vi "FlexMag - 24-03-2023.vi"() -> ()   [LabVIEW 2018] (continued)
            n18652 = local write "CH2_Motor DO"(w23090) -> ()
            n18653 = local write "CH3_Motor DO"(w23090) -> ()
            n18654 = local write "CH4_Motor DO"(w23090) -> ()
            n18655 = local write "step count"(0.0 ("step count")) -> ()
            n18656 = local write "forward roll"(FALSE ("forward roll")) -> ()
            n18657 = Wait (ms)(milliseconds to wait=u32 300) -> ()  [unwired: 1 out]
          }
        }
      }
      frame 2 {
        # "backward roll"
        n18658 = stacked-sequence {
          tunnel: w23093 -> [w23094 _ _ _ _ _ w23153 w23163 _]
          frame #0 {
            n18659 = Wait (ms)(milliseconds to wait=u32 100) -> ()  [unwired: 1 out]
            n18660 = case shown="0, Default" w23094 {
              frame 0, Default {
                n18661 = local write "roll error"(TRUE ("roll error")) -> ()
                n18662 = local write "Warning Message"("Choose Cassette Position !" ("Warning Message")) -> ()
                n18663 = Wait (ms)(milliseconds to wait=u32 100) -> ()  [unwired: 1 out]
              }
              frame 1 {
                n18664 = local read "CH1_SRV1_Piston_For_DI"() -> (w23099:bool)
                n18665 = case shown="False" w23099 {
                  frame False {
                    n18666 = local write "roll error"(TRUE ("roll error")) -> ()
                    n18667 = Wait (ms)(milliseconds to wait=u32 100) -> ()  [unwired: 1 out]
                  }
                  frame True {
                  }
                }
              }
              frame 2 {
                n18668 = local read "CH2_SRV1_Piston_For_DI"() -> (w23102:bool)
                n18669 = case shown="False" w23102 {
                  frame False {
                    n18670 = local write "roll error"(TRUE ("roll error")) -> ()
                    n18671 = Wait (ms)(milliseconds to wait=u32 100) -> ()  [unwired: 1 out]
                  }
                  frame True {
                  }
                }
              }
              frame 3 {
                n18672 = local read "CH3_SRV1_Piston_For_DI"() -> (w23105:bool)
                n18673 = case shown="False" w23105 {
                  frame False {
                    n18674 = local write "roll error"(TRUE ("roll error")) -> ()
                    n18675 = Wait (ms)(milliseconds to wait=u32 100) -> ()  [unwired: 1 out]
                  }
                  frame True {
                  }
                }
              }
              frame 4 {
                n18676 = local read "CH4_SRV1_Piston_For_DI"() -> (w23108:bool)
                n18677 = case shown="False" w23108 {
                  frame False {
                    n18678 = local write "roll error"(TRUE ("roll error")) -> ()
                    n18679 = Wait (ms)(milliseconds to wait=u32 100) -> ()  [unwired: 1 out]
                  }
                  frame True {
                  }
                }
              }
            }
          }
          frame #1 {
            n18680 = flat-sequence {
              frame #0 {
                n18681 = local write "Roll Forw"(FALSE ("Roll Forw")) -> ()
              }
              frame #1 {
                n18682 = Wait (ms)(milliseconds to wait=u32 300) -> ()  [unwired: 1 out]
              }
              frame #2 {
                n18683 = local write "TC parameter set"(TRUE ("TC parameter set")) -> ()
              }
              frame #3 {
                n18684 = Wait (ms)(milliseconds to wait=u32 300) -> ()  [unwired: 1 out]
              }
            }
            n18685 = disable-structure shown="Disabled" {
              frame Disabled {
                n18686 = local read "lap number right actual"() -> (w23114:dbl)
                n18687 = local write "lap number left target"(w23114) -> ()
              }
              frame Enabled {
              }
            }
            n18688 = local write "lap number left actual"(0.0 ("lap number left actual")) -> ()
            n18689 = local write "lap number right actual"(0.0 ("lap number left actual")) -> ()
            n18690 = local read "step count"() -> (w23112:dbl)
            n18691 = local write "step count 2"(w23112) -> ()
          }
          frame #2 {
            n18692 = local read "back roll"() -> (w23119:bool)
            n18693 = case shown="True" w23119 {
              frame False {
              }
              frame True {
                n18694 = while {
                  i -> [w23125]
                  stop <- w23123 stop-if-true
                  n18695 = Wait Until Next ms Multiple(millisecond multiple=u32 300) -> ()  [unwired: 1 out]
                  n18696 = local read "TC parameter set"() -> (w23129:bool)
                  n18697 = local read "back roll"() -> (w23121:bool)
                  n18698 = local read "ABORT"() -> (w23127:bool)
                  n18699 = Not(x=w23129) -> (.not. x?=w23126:bool)
                  n18700 = Not(x=w23121) -> (.not. x?=w23120:bool)
                  n18701 = Greater Or Equal?(x=w23125, y=u32 400 ("millisecond multiple")) -> (x >= y?=w23122:bool)
                  n18702 = Compound Arithmetic op=OR(w23122, w23126, w23127, w23120) -> (w23123:bool)
                  n18703 = local write "roll error"(w23122) -> ()
                }
              }
            }
          }
          frame #3 {
            n18704 = local read "back roll"() -> (w23130:bool)
            n18705 = case shown="True" w23130 {
              frame False {
              }
              frame True {
                n18706 = flat-sequence {
                  frame #0 {
                    n18707 = disable-structure shown="Enabled" {
                      disable-tunnel: [w23134 sgl 0.1 ("TC1_overspeed_value")] -> w23131
                      frame Disabled {
                        n18708 = local read "output_pid"() -> (w23134:dbl)
                      }
                      frame Enabled {
                      }
                    }
                    n18709 = local read "tension value"() -> (w23133:dbl)
                    n18710 = local write "TC2_set_value"(w23133) -> ()
                    n18711 = local write "TC1_overspeed_value"(w23131) -> ()
                    n18712 = local write "current voltage"(w23131) -> ()
                    n18713 = Wait (ms)(milliseconds to wait=u32 1000) -> ()  [unwired: 1 out]
                  }
                  frame #1 {
                    n18714 = local write "TC1_overspeed_set"(TRUE ("TC2 Set moxa")) -> ()
                    n18715 = local write "TC2_auto_set"(TRUE ("TC1_set")) -> ()
                  }
                  frame #2 {
                    n18716 = local write "TC2_overspeed_value"(sgl 0.0 ("TC2_set_value")) -> ()
                    n18717 = local write "TC1_set_value"(sgl 0.0 ("TC2_set_value")) -> ()
                    n18718 = Wait (ms)(milliseconds to wait=u32 2000) -> ()  [unwired: 1 out]
                  }
                  frame #3 {
                    n18719 = local write "TC2_overspeed_set"(TRUE ("TC2_auto_set")) -> ()
                    n18720 = local write "TC1_auto_set"(TRUE ("TC2_auto_set")) -> ()
                  }
                }
              }
            }
          }
          frame #4 {
            n18721 = local read "back roll"() -> (w23143:bool)
            n18722 = case shown="True" w23143 {
              frame False {
              }
              frame True {
                n18723 = flat-sequence {
                  frame #0 {
                    w23145 = FALSE ("CH1_SRV_Direction_Clockwise_DO")
                    n18724 = Wait (ms)(milliseconds to wait=u32 100) -> ()  [unwired: 1 out]
                    n18725 = local write "CH1_SRV_Direction_Clockwise_DO"(w23145) -> ()
                    n18726 = local write "CH2_SRV_Direction_Clockwise_DO"(w23145) -> ()
                    n18727 = local write "CH3_SRV_Direction_Clockwise_DO"(w23145) -> ()
                    n18728 = local write "CH4_SRV_Direction_Clockwise_DO"(w23145) -> ()
                    n18729 = disable-structure shown="Disabled" {
                      frame Disabled {
                        n18730 = local write "setpoint"(0.1 ("setpoint")) -> ()
                      }
                      frame Enabled {
                      }
                    }
                  }
                  frame #1 {
                    n18731 = Wait (ms)(milliseconds to wait=u32 3000) -> ()  [unwired: 1 out]
                  }
                }
              }
            }
          }
          frame #5 {
            n18732 = local read "back roll"() -> (w23148:bool)
            n18733 = case shown="True" w23148 {
              frame False {
              }
              frame True {
                n18734 = disable-structure shown="Disabled" {
                  frame Disabled {
                    w23151 = 0.1 ("lower limit")
                    n18735 = Bundle("lower limit"=w23151, "lower limit"=w23151) -> (w23152:cluster{"lower limit":dbl, "lower limit":dbl})  [unwired: 1 in]
                    n18736 = local write "output range"(w23152) -> ()
                  }
                  frame Enabled {
                  }
                }
                n18737 = local write "Tension_Controllers_Start/Stop DO"(TRUE ("CH1_SRV_Direction_Clockwise_DO")) -> ()
                n18738 = Wait (ms)(milliseconds to wait=u32 100) -> ()  [unwired: 1 out]
              }
            }
          }
          frame #6 {
            n18739 = local read "back roll"() -> (w23154:bool)
            n18740 = case shown="True" w23154 {
              tunnel: w23153 -> [_ w23157]
              frame False {
              }
              frame True {
                n18741 = case shown="1" w23157 {
                  frame 0, Default {
                    n18742 = local write "roll error"(TRUE ("roll error")) -> ()
                  }
                  frame 1 {
                    n18743 = local write "CH1_Motor DO"(TRUE ("CH1_Motor DO")) -> ()
                  }
                  frame 2 {
                    n18744 = local write "CH2_Motor DO"(TRUE ("CH1_Motor DO")) -> ()
                  }
                  frame 3 {
                    n18745 = local write "CH3_Motor DO"(TRUE ("CH1_Motor DO")) -> ()
                  }
                  frame 4 {
                    n18746 = local write "CH4_Motor DO"(TRUE ("CH1_Motor DO")) -> ()
                  }
                }
                n18747 = local write "QR continuous mode"(TRUE ("QR continuous mode")) -> ()
                n18748 = local write "pid output"(TRUE ("pid output")) -> ()
              }
            }
          }
          frame #7 {
            n18749 = local read "back roll"() -> (w23164:bool)
            n18750 = case shown="True" w23164 {
              tunnel: w23163 -> [_ w23165]
              frame False {
              }
              frame True {
                n18751 = case shown="4" w23165 {
                  frame 0, Default {
                    n18752 = local write "roll error"(TRUE ("roll error")) -> ()
                  }
                  frame 1 {
                    n18753 = while {
                      i -> [w23187]
                      stop <- w23197 stop-if-true
                      n18754 = local read "CH1_SRV2_COUNTER_DI"() -> (w23193:bool)
                      n18755 = local read "Ch1_srv1_counter DI"() -> (w23185:bool)
                      n18756 = Wait Until Next ms Multiple(millisecond multiple=u32 100) -> ()  [unwired: 1 out]
                      n18757 = Greater Or Equal?(x=w23187, y=200) -> (x >= y?=w23188:bool)
                      n18758 = feedback #330() -> (w23194:bool)  [unwired: 1 in]
                      n18759 = feedback-in #330(w23193) -> ()
                      n18760 = feedback #331() -> (w23184:bool)  [unwired: 1 in]
                      n18761 = feedback-in #331(w23185) -> ()
                      n18762 = case shown="True" w23188 {
                        tunnel: [FALSE ("backroll stop cmd") w23204] -> w23190
                        frame False {
                        }
                        frame True {
                          n18763 = local read "backroll stop cmd"() -> (w23204:bool)
                        }
                      }
                      n18764 = Implies(1:w23193, 2:w23194) -> (0:w23195:bool)
                      n18765 = Implies(1:w23185, 2:w23184) -> (0:w23183:bool)
                      n18766 = Not(x=w23195) -> (.not. x?=w23192:bool)
                      n18767 = Not(x=w23183) -> (.not. x?=w23182:bool)
                      n18768 = local read "max rotation number"() -> (w23177:dbl)
                      n18769 = case shown="True" w23192 {
                        frame False {
                        }
                        frame True {
                          n18770 = local read "output range"() -> (w23205:cluster{"output high":dbl, "output low":dbl})
                          n18771 = local read "lap number right actual"() -> (w23212:dbl)
                          n18772 = Unbundle By Name(w23205) -> ("output high"=w23207:dbl, "output low"=w23210:dbl)
                          n18773 = Increment(x=w23212) -> (x+1=w23211:dbl)
                          n18774 = local read "decreasing voltage"() -> (w23206:dbl)
                          n18775 = local write "lap number right actual"(w23211) -> ()
                          n18776 = Subtract(x=w23207, y=w23206) -> (x-y=w23209:dbl)
                          n18777 = Bundle(w23209, "output low"=w23210) -> (w23208:cluster{dbl, "output low":dbl})  [unwired: 1 in]
                          n18778 = local write "output range"(w23208) -> ()
                        }
                      }
                      n18779 = case shown="True" w23182 {
                        frame False {
                        }
                        frame True {
                          n18780 = local read "lap number left actual"() -> (w23202:dbl)
                          n18781 = Increment(x=w23202) -> (x+1=w23201:dbl)
                          n18782 = local write "lap number left actual"(w23201) -> ()
                        }
                      }
                      n18783 = local read "lap number right actual"() -> (w23186:dbl)
                      n18784 = local read "lap number left actual"() -> (w23181:dbl)
                      n18785 = local read "abort ch1"() -> (w23191:bool)
                      n18786 = local read "back roll"() -> (w23200:bool)
                      n18787 = Greater Or Equal?(x=w23181, y=w23177) -> (x >= y?=w23179:bool)
                      n18788 = Greater Or Equal?(x=w23186, y=w23177) -> (x >= y?=w23180:bool)
                      n18789 = Not(x=w23200) -> (.not. x?=w23199:bool)
                      n18790 = Or(x=w23180, y=w23179) -> (x .or. y?=w23178:bool)
                      n18791 = Compound Arithmetic op=OR(w23191, w23199, w23190, w23178) -> (w23197:bool)
                      n18792 = Not(x=w23197) -> (.not. x?=w23198:bool)
                      n18793 = local write "CH1_Motor DO"(w23198) -> ()
                    }
                    n18794 = while {
                      stop <- w23173 stop-if-true
                      n18795 = stacked-sequence {
                        frame #0 {
                          n18796 = local read "output_pid"() -> (w23174:dbl)
                          n18797 = Wait (ms)(milliseconds to wait=u32 25) -> ()  [unwired: 1 out]
                          n18798 = local write "TC1_overspeed_value"(w23174) -> ()
                          n18799 = local write "current voltage"(w23174) -> ()
                        }
                        frame #1 {
                          n18800 = local write "TC1_overspeed_set"(TRUE ("TC2_overspeed_set")) -> ()
                        }
                      }
                      n18801 = local read "CH1_Motor DO"() -> (w23168:bool)
                      n18802 = local read "back roll"() -> (w23171:bool)
                      n18803 = local read "set speed (ms)"() -> (w23169:u32)
                      n18804 = local read "abort ch1"() -> (w23172:bool)
                      n18805 = Not(x=w23171) -> (.not. x?=w23170:bool)
                      n18806 = Not(x=w23168) -> (.not. x?=w23167:bool)
                      n18807 = Compound Arithmetic op=OR(w23167, w23172, w23170) -> (w23173:bool)
                      n18808 = Wait Until Next ms Multiple(millisecond multiple=w23169) -> ()  [unwired: 1 out]
                    }
                  }
                  frame 2 {
                    n18809 = while {
                      i -> [w23234]
                      stop <- w23243 stop-if-true
                      n18810 = local read "CH2_SRV2_COUNTER_DI"() -> (w23239:bool)
                      n18811 = Greater Or Equal?(x=w23234, y=200) -> (x >= y?=w23233:bool)
                      n18812 = case shown="True" w23233 {
                        tunnel: [FALSE ("backroll stop cmd") w23250] -> w23236
                        frame False {
                        }
                        frame True {
                          n18813 = local read "backroll stop cmd"() -> (w23250:bool)
                        }
                      }
                      n18814 = local read "Ch2_srv1_counter DI"() -> (w23228:bool)
                      n18815 = feedback #332() -> (w23240:bool)  [unwired: 1 in]
                      n18816 = feedback-in #332(w23239) -> ()
                      n18817 = Implies(1:w23239, 2:w23240) -> (0:w23241:bool)
                      n18818 = Not(x=w23241) -> (.not. x?=w23238:bool)
                      n18819 = local read "max rotation number"() -> (w23223:dbl)
                      n18820 = case shown="True" w23238 {
                        frame False {
                        }
                        frame True {
                          n18821 = local read "lap number right actual"() -> (w23258:dbl)
                          n18822 = local read "output range"() -> (w23251:cluster{"output high":dbl, "output low":dbl})
                          n18823 = Unbundle By Name(w23251) -> ("output high"=w23253:dbl, "output low"=w23256:dbl)
                          n18824 = Increment(x=w23258) -> (x+1=w23257:dbl)
                          n18825 = local write "lap number right actual"(w23257) -> ()
                          n18826 = local read "decreasing voltage"() -> (w23252:dbl)
                          n18827 = Subtract(x=w23253, y=w23252) -> (x-y=w23255:dbl)
                          n18828 = Bundle(w23255, "output low"=w23256) -> (w23254:cluster{dbl, "output low":dbl})  [unwired: 1 in]
                          n18829 = local write "output range"(w23254) -> ()
                        }
                      }
                      n18830 = feedback #333() -> (w23229:bool)  [unwired: 1 in]
                      n18831 = feedback-in #333(w23228) -> ()
                      n18832 = Implies(1:w23228, 2:w23229) -> (0:w23230:bool)
                      n18833 = Not(x=w23230) -> (.not. x?=w23231:bool)
                      n18834 = local read "lap number right actual"() -> (w23232:dbl)
                      n18835 = case shown="True" w23231 {
                        frame False {
                        }
                        frame True {
                          n18836 = local read "lap number left actual"() -> (w23248:dbl)
                          n18837 = Increment(x=w23248) -> (x+1=w23247:dbl)
                          n18838 = local write "lap number left actual"(w23247) -> ()
                        }
                      }
                      n18839 = local read "lap number left actual"() -> (w23227:dbl)
                      n18840 = Greater Or Equal?(x=w23232, y=w23223) -> (x >= y?=w23226:bool)
                      n18841 = local read "abort ch2"() -> (w23237:bool)
                      n18842 = local read "back roll"() -> (w23246:bool)
                      n18843 = Greater Or Equal?(x=w23227, y=w23223) -> (x >= y?=w23225:bool)
                      n18844 = Or(x=w23226, y=w23225) -> (x .or. y?=w23224:bool)
                      n18845 = Not(x=w23246) -> (.not. x?=w23245:bool)
                      n18846 = Compound Arithmetic op=OR(w23237, w23245, w23236, w23224) -> (w23243:bool)
                      n18847 = Not(x=w23243) -> (.not. x?=w23244:bool)
                      n18848 = local write "CH2_Motor DO"(w23244) -> ()
                      n18849 = Wait Until Next ms Multiple(millisecond multiple=u32 100) -> ()  [unwired: 1 out]
                    }
                    n18850 = while {
                      stop <- w23219 stop-if-true
                      n18851 = stacked-sequence {
                        frame #0 {
                          n18852 = local read "output_pid"() -> (w23220:dbl)
                          n18853 = Wait (ms)(milliseconds to wait=u32 25) -> ()  [unwired: 1 out]
                          n18854 = local write "TC1_overspeed_value"(w23220) -> ()
                          n18855 = local write "current voltage"(w23220) -> ()
                        }
                        frame #1 {
                          n18856 = local write "TC1_overspeed_set"(TRUE ("TC2_overspeed_set")) -> ()
                        }
                      }
                      n18857 = local read "CH2_Motor DO"() -> (w23214:bool)
                      n18858 = local read "back roll"() -> (w23217:bool)
                      n18859 = local read "set speed (ms)"() -> (w23215:u32)
                      n18860 = local read "abort ch2"() -> (w23218:bool)
                      n18861 = Not(x=w23217) -> (.not. x?=w23216:bool)
                      n18862 = Not(x=w23214) -> (.not. x?=w23213:bool)
                      n18863 = Compound Arithmetic op=OR(w23213, w23218, w23216) -> (w23219:bool)
                      n18864 = Wait Until Next ms Multiple(millisecond multiple=w23215) -> ()  [unwired: 1 out]
                    }
                  }
                  frame 3 {
                    n18865 = while {
                      i -> [w23284]
                      stop <- w23279 stop-if-true
                      n18866 = local read "CH3_SRV2_COUNTER_DI"() -> (w23287:bool)
                      n18867 = Greater Or Equal?(x=w23284, y=200) -> (x >= y?=w23283:bool)
                      n18868 = case shown="True" w23283 {
                        tunnel: [FALSE ("backroll stop cmd") w23296] -> w23280
                        frame False {
                        }
                        frame True {
                          n18869 = local read "backroll stop cmd"() -> (w23296:bool)
                        }
                      }
                      n18870 = feedback #334() -> (w23288:bool)  [unwired: 1 in]
                      n18871 = feedback-in #334(w23287) -> ()
                      n18872 = local read "Ch3_srv1_counter DI"() -> (w23277:bool)
                      n18873 = Implies(1:w23287, 2:w23288) -> (0:w23289:bool)
                      n18874 = Not(x=w23289) -> (.not. x?=w23286:bool)
                      n18875 = case shown="True" w23286 {
                        frame False {
                        }
                        frame True {
                          n18876 = local read "output range"() -> (w23302:cluster{"output high":dbl, "output low":dbl})
                          n18877 = local read "lap number right actual"() -> (w23304:dbl)
                          n18878 = Unbundle By Name(w23302) -> ("output high"=w23300:dbl, "output low"=w23297:dbl)
                          n18879 = Increment(x=w23304) -> (x+1=w23303:dbl)
                          n18880 = local read "decreasing voltage"() -> (w23301:dbl)
                          n18881 = local write "lap number right actual"(w23303) -> ()
                          n18882 = Subtract(x=w23300, y=w23301) -> (x-y=w23298:dbl)
                          n18883 = Bundle(w23298, "output low"=w23297) -> (w23299:cluster{dbl, "output low":dbl})  [unwired: 1 in]
                          n18884 = local write "output range"(w23299) -> ()
                        }
                      }
                      n18885 = local read "max rotation number"() -> (w23269:dbl)
                      n18886 = local read "lap number right actual"() -> (w23278:dbl)
                      n18887 = feedback #335() -> (w23276:bool)  [unwired: 1 in]
                      n18888 = feedback-in #335(w23277) -> ()
                      n18889 = Implies(1:w23277, 2:w23276) -> (0:w23275:bool)
                      n18890 = Not(x=w23275) -> (.not. x?=w23274:bool)
                      n18891 = case shown="True" w23274 {
                        frame False {
                        }
                        frame True {
                          n18892 = local read "lap number left actual"() -> (w23294:dbl)
                          n18893 = Increment(x=w23294) -> (x+1=w23293:dbl)
                          n18894 = local write "lap number left actual"(w23293) -> ()
                        }
                      }
                      n18895 = local read "lap number left actual"() -> (w23273:dbl)
                      n18896 = Greater Or Equal?(x=w23278, y=w23269) -> (x >= y?=w23271:bool)
                      n18897 = local read "abort ch3"() -> (w23282:bool)
                      n18898 = local read "back roll"() -> (w23292:bool)
                      n18899 = Greater Or Equal?(x=w23273, y=w23269) -> (x >= y?=w23272:bool)
                      n18900 = Not(x=w23292) -> (.not. x?=w23281:bool)
                      n18901 = Or(x=w23271, y=w23272) -> (x .or. y?=w23270:bool)
                      n18902 = Compound Arithmetic op=OR(w23282, w23281, w23280, w23270) -> (w23279:bool)
                      n18903 = Not(x=w23279) -> (.not. x?=w23291:bool)
                      n18904 = local write "CH3_Motor DO"(w23291) -> ()
                      n18905 = Wait Until Next ms Multiple(millisecond multiple=u32 100) -> ()  [unwired: 1 out]
                    }
                    n18906 = while {
                      stop <- w23265 stop-if-true
                      n18907 = stacked-sequence {
                        frame #0 {
                          n18908 = local read "output_pid"() -> (w23266:dbl)
                          n18909 = Wait (ms)(milliseconds to wait=u32 25) -> ()  [unwired: 1 out]
                          n18910 = local write "TC1_overspeed_value"(w23266) -> ()
                          n18911 = local write "current voltage"(w23266) -> ()
                        }
                        frame #1 {
                          n18912 = local write "TC1_overspeed_set"(TRUE ("TC2_overspeed_set")) -> ()
                        }
                      }
                      n18913 = local read "CH3_Motor DO"() -> (w23260:bool)
                      n18914 = local read "back roll"() -> (w23263:bool)
                      n18915 = local read "set speed (ms)"() -> (w23261:u32)
                      n18916 = local read "abort ch3"() -> (w23264:bool)
                      n18917 = Not(x=w23263) -> (.not. x?=w23262:bool)
                      n18918 = Not(x=w23260) -> (.not. x?=w23259:bool)
                      n18919 = Compound Arithmetic op=OR(w23259, w23264, w23262) -> (w23265:bool)
                      n18920 = Wait Until Next ms Multiple(millisecond multiple=w23261) -> ()  [unwired: 1 out]
                    }
                  }
                  frame 4 {
                    n18921 = while {
                      i -> [w23325]
                      stop <- w23335 stop-if-true
                      n18922 = local read "CH4_SRV2_COUNTER_DI"() -> (w23331:bool)
                      n18923 = feedback #336() -> (w23332:bool)  [unwired: 1 in]
                      n18924 = feedback-in #336(w23331) -> ()
                      n18925 = local read "Ch4_srv1_counter DI"() -> (w23321:bool)
                      n18926 = Implies(1:w23331, 2:w23332) -> (0:w23333:bool)
                      n18927 = Not(x=w23333) -> (.not. x?=w23330:bool)
                      n18928 = Greater Or Equal?(x=w23325, y=200) -> (x >= y?=w23326:bool)
                      n18929 = case shown="True" w23330 {
                        frame False {
                        }
                        frame True {
                          n18930 = local read "output range"() -> (w23348:cluster{"output high":dbl, "output low":dbl})
                          n18931 = local read "lap number right actual"() -> (w23350:dbl)
                          n18932 = Unbundle By Name(w23348) -> ("output high"=w23346:dbl, "output low"=w23343:dbl)
                          n18933 = local read "decreasing voltage"() -> (w23347:dbl)
                          n18934 = Increment(x=w23350) -> (x+1=w23349:dbl)
                          n18935 = local write "lap number right actual"(w23349) -> ()
                          n18936 = Subtract(x=w23346, y=w23347) -> (x-y=w23344:dbl)
                          n18937 = Bundle(w23344, "output low"=w23343) -> (w23345:cluster{dbl, "output low":dbl})  [unwired: 1 in]
                          n18938 = local write "output range"(w23345) -> ()
                        }
                      }
                      n18939 = local read "max rotation number"() -> (w23315:dbl)
                      n18940 = case shown="True" w23326 {
                        tunnel: [FALSE w23342] -> w23328
                        frame False {
                        }
                        frame True {
                          n18941 = local read "backroll stop cmd"() -> (w23342:bool)
                        }
                      }
                      n18942 = feedback #337() -> (w23322:bool)  [unwired: 1 in]
                      n18943 = feedback-in #337(w23321) -> ()
                      n18944 = Implies(1:w23321, 2:w23322) -> (0:w23323:bool)
                      n18945 = Not(x=w23323) -> (.not. x?=w23320:bool)
                      n18946 = case shown="True" w23320 {
                        frame False {
                        }
                        frame True {
                          n18947 = local read "lap number left actual"() -> (w23339:dbl)
                          n18948 = Increment(x=w23339) -> (x+1=w23340:dbl)
                          n18949 = local write "lap number left actual"(w23340) -> ()
                        }
                      }
                      n18950 = local read "lap number right actual"() -> (w23324:dbl)
                      n18951 = local read "lap number left actual"() -> (w23319:dbl)
                      n18952 = Greater Or Equal?(x=w23324, y=w23315) -> (x >= y?=w23318:bool)
                      n18953 = Greater Or Equal?(x=w23319, y=w23315) -> (x >= y?=w23317:bool)
                      n18954 = local read "abort ch4"() -> (w23329:bool)
                      n18955 = local read "back roll"() -> (w23338:bool)
                      n18956 = Or(x=w23318, y=w23317) -> (x .or. y?=w23316:bool)
                      n18957 = Not(x=w23338) -> (.not. x?=w23337:bool)
                      n18958 = Compound Arithmetic op=OR(w23329, w23337, w23328, w23316) -> (w23335:bool)
                      n18959 = Not(x=w23335) -> (.not. x?=w23336:bool)
                      n18960 = local write "CH4_Motor DO"(w23336) -> ()
                      n18961 = Wait Until Next ms Multiple(millisecond multiple=u32 100) -> ()  [unwired: 1 out]
                    }
                    n18962 = while {
                      stop <- w23311 stop-if-true
                      n18963 = stacked-sequence {
                        frame #0 {
                          n18964 = local read "output_pid"() -> (w23312:dbl)
                          n18965 = Wait (ms)(milliseconds to wait=u32 25) -> ()  [unwired: 1 out]
                          n18966 = local write "TC1_overspeed_value"(w23312) -> ()
                          n18967 = local write "current voltage"(w23312) -> ()
                        }
                        frame #1 {
                          n18968 = local write "TC1_overspeed_set"(TRUE ("TC2_overspeed_set")) -> ()
                        }
                      }
                      n18969 = local read "CH4_Motor DO"() -> (w23306:bool)
                      n18970 = local read "back roll"() -> (w23309:bool)
                      n18971 = local read "abort ch4"() -> (w23310:bool)
                      n18972 = local read "set speed (ms)"() -> (w23307:u32)
                      n18973 = Not(x=w23306) -> (.not. x?=w23305:bool)
                      n18974 = Not(x=w23309) -> (.not. x?=w23308:bool)
                      n18975 = Compound Arithmetic op=OR(w23305, w23310, w23308) -> (w23311:bool)
                      n18976 = Wait Until Next ms Multiple(millisecond multiple=w23307) -> ()  [unwired: 1 out]
                    }
                  }
                }
              }
            }
          }
          frame #8 {
            w23352 = FALSE ("forward roll")
            n18977 = local write "Tension_Controllers_Start/Stop DO"(w23352) -> ()
            n18978 = local write "CH1_Motor DO"(w23352) -> ()
            n18979 = local write "CH2_Motor DO"(w23352) -> ()
            n18980 = local write "CH3_Motor DO"(w23352) -> ()
            n18981 = local write "CH4_Motor DO"(w23352) -> ()
            n18982 = local write "step count"(0.0 ("step count")) -> ()
            n18983 = local write "back roll"(FALSE ("forward roll")) -> ()
            n18984 = Wait (ms)(milliseconds to wait=u32 300) -> ()  [unwired: 1 out]
          }
        }
      }
      frame 3 {
        n18985 = stacked-sequence {
          tunnel: w23355 -> [_ _ _ _ _ w23388 w23397 _ _ _ _ _ w23551 w23560]
          frame #0 {
            n18986 = flat-sequence {
              frame #0 {
                n18987 = local write "Roll Forw"(FALSE ("Roll Forw")) -> ()
              }
              frame #1 {
                n18988 = Wait (ms)(milliseconds to wait=u32 300) -> ()  [unwired: 1 out]
              }
              frame #2 {
                n18989 = local write "TC parameter set"(TRUE ("TC parameter set")) -> ()
              }
              frame #3 {
                n18990 = Wait (ms)(milliseconds to wait=u32 300) -> ()  [unwired: 1 out]
              }
            }
          }
          frame #1 {
            n18991 = local read "position"() -> (w23360:bool)
            n18992 = case shown="True" w23360 {
              frame False {
              }
              frame True {
                n18993 = while {
                  i -> [w23366]
                  stop <- w23364 stop-if-true
                  n18994 = Wait Until Next ms Multiple(millisecond multiple=u32 300) -> ()  [unwired: 1 out]
                  n18995 = local read "TC parameter set"() -> (w23370:bool)
                  n18996 = local read "position"() -> (w23362:bool)
                  n18997 = local read "ABORT"() -> (w23368:bool)
                  n18998 = Not(x=w23370) -> (.not. x?=w23367:bool)
                  n18999 = Not(x=w23362) -> (.not. x?=w23361:bool)
                  n19000 = Greater Or Equal?(x=w23366, y=u32 400 ("millisecond multiple")) -> (x >= y?=w23363:bool)
                  n19001 = Compound Arithmetic op=OR(w23363, w23367, w23368, w23361) -> (w23364:bool)
                  n19002 = local write "roll error"(w23363) -> ()
                }
              }
            }
          }
          frame #2 {
            n19003 = local read "position"() -> (w23371:bool)
            n19004 = case shown="True" w23371 {
              frame False {
              }
              frame True {
                n19005 = flat-sequence {
                  frame #0 {
                    w23372 = sgl 0.5 ("TC2_overspeed_value")
                    n19006 = local read "tension value"() -> (w23374:dbl)
                    n19007 = Wait (ms)(milliseconds to wait=u32 300) -> ()  [unwired: 1 out]
                    n19008 = local write "TC2_set_value"(w23374) -> ()
                    n19009 = local write "TC1_overspeed_value"(w23372) -> ()
                    n19010 = local write "current voltage"(w23372) -> ()
                  }
                  frame #1 {
                    n19011 = local write "TC1_overspeed_set"(TRUE ("TC2 Set moxa")) -> ()
                    n19012 = local write "TC2_auto_set"(TRUE ("TC1_set")) -> ()
                  }
                  frame #2 {
                    n19013 = local write "TC2_overspeed_value"(sgl 0.0 ("TC1_set_value")) -> ()
                    n19014 = local write "TC1_set_value"(sgl 0.0 ("TC1_set_value")) -> ()
                    n19015 = Wait (ms)(milliseconds to wait=u32 300) -> ()  [unwired: 1 out]
                  }
                  frame #3 {
                    n19016 = local write "TC2_overspeed_set"(TRUE ("TC1_auto_set")) -> ()
                    n19017 = local write "TC1_auto_set"(TRUE ("TC1_auto_set")) -> ()
                  }
                }
              }
            }
          }
          frame #3 {
            n19018 = local read "position"() -> (w23382:bool)
            n19019 = case shown="True" w23382 {
              frame False {
              }
              frame True {
                w23384 = FALSE ("CH1_SRV_Direction_Clockwise_DO")
                n19020 = local write "CH1_SRV_Direction_Clockwise_DO"(w23384) -> ()
                n19021 = local write "CH2_SRV_Direction_Clockwise_DO"(w23384) -> ()
                n19022 = local write "CH3_SRV_Direction_Clockwise_DO"(w23384) -> ()
                n19023 = local write "CH4_SRV_Direction_Clockwise_DO"(w23384) -> ()
                n19024 = Wait (ms)(milliseconds to wait=u32 100) -> ()  [unwired: 1 out]
              }
            }
          }
          frame #4 {
            n19025 = local read "position"() -> (w23385:bool)
            n19026 = case shown="True" w23385 {
              frame False {
              }
              frame True {
                n19027 = local write "Tension_Controllers_Start/Stop DO"(TRUE ("CH1_SRV_Direction_Clockwise_DO")) -> ()
                n19028 = Wait (ms)(milliseconds to wait=u32 100) -> ()  [unwired: 1 out]
              }
            }
          }
          frame #5 {
            n19029 = local read "position"() -> (w23389:bool)
            n19030 = case shown="True" w23389 {
              tunnel: w23388 -> [_ w23390]
              frame False {
              }
              frame True {
                n19031 = Wait (ms)(milliseconds to wait=u32 100) -> ()  [unwired: 1 out]
                n19032 = case shown="2" w23390 {
                  frame 0, Default {
                    n19033 = local write "roll error"(TRUE ("roll error")) -> ()
                  }
                  frame 1 {
                    n19034 = local write "CH1_Motor DO"(TRUE ("CH1_Motor DO")) -> ()
                  }
                  frame 2 {
                    n19035 = local write "CH2_Motor DO"(TRUE ("CH1_Motor DO")) -> ()
                  }
                  frame 3 {
                    n19036 = local write "CH3_Motor DO"(TRUE ("CH1_Motor DO")) -> ()
                  }
                  frame 4 {
                    n19037 = local write "CH4_Motor DO"(TRUE ("CH1_Motor DO")) -> ()
                  }
                }
              }
            }
          }
          frame #6 {
            n19038 = local read "position"() -> (w23398:bool)
            n19039 = case shown="True" w23398 {
              tunnel: w23397 -> [_ w23399]
              frame False {
              }
              frame True {
                n19040 = case shown="3" w23399 {
                  frame 0, Default {
                  }
                  frame 1 {
                    n19041 = local read "Ch1_srv1_counter DI"() -> (w23400:bool)
                    n19042 = case shown="False" w23400 {
                      frame False {
                        n19043 = stacked-sequence {
                          frame #0 {
                            n19044 = while {
                              stop <- w23404 stop-if-true
                              n19045 = local read "Ch1_srv1_counter DI"() -> (w23406:bool)
                              n19046 = Wait Until Next ms Multiple(millisecond multiple=u32 100) -> ()  [unwired: 1 out]
                              n19047 = case shown="True" w23406 {
                                tunnel: [FALSE TRUE] -> w23402
                                frame False {
                                }
                                frame True {
                                }
                              }
                              n19048 = local read "position"() -> (w23405:bool)
                              n19049 = Not(x=w23405) -> (.not. x?=w23403:bool)
                              n19050 = Or(x=w23402, y=w23403) -> (x .or. y?=w23404:bool)
                            }
                          }
                          frame #1 {
                            n19051 = while {
                              stop <- w23409 stop-if-true
                              n19052 = local read "Ch1_srv1_counter DI"() -> (w23415:bool)
                              n19053 = Wait Until Next ms Multiple(millisecond multiple=u32 100) -> ()  [unwired: 1 out]
                              n19054 = case shown="False" w23415 {
                                tunnel: [TRUE FALSE] -> w23412
                                frame False {
                                n19055 = local write "CH1_Motor DO"(FALSE ("CH1_Motor DO")) -> ()
                                }
                                frame True {
                                }
                              }
                              n19056 = local read "position"() -> (w23414:bool)
                              n19057 = Not(x=w23414) -> (.not. x?=w23413:bool)
                              n19058 = Or(x=w23412, y=w23413) -> (x .or. y?=w23409:bool)
                              n19059 = Not(x=w23409) -> (.not. x?=w23410:bool)
                              n19060 = local write "CH1_Motor DO"(w23410) -> ()
                            }
                          }
                        }
                      }
                      frame True {
                        n19061 = while {
                          stop <- w23421 stop-if-true
                          n19062 = local read "Ch1_srv1_counter DI"() -> (w23419:bool)
                          n19063 = Wait Until Next ms Multiple(millisecond multiple=u32 100) -> ()  [unwired: 1 out]
                          n19064 = case shown="False" w23419 {
                            tunnel: [TRUE FALSE] -> w23423
                            frame False {
                              n19065 = local write "CH1_Motor DO"(FALSE ("CH1_Motor DO")) -> ()
                            }
                            frame True {
                            }
                          }
                          n19066 = local read "position"() -> (w23425:bool)
                          n19067 = Not(x=w23425) -> (.not. x?=w23424:bool)
                          n19068 = Or(x=w23423, y=w23424) -> (x .or. y?=w23421:bool)
                          n19069 = Not(x=w23421) -> (.not. x?=w23422:bool)
                          n19070 = local write "CH1_Motor DO"(w23422) -> ()
                        }
                      }
                    }
                  }
                  frame 2 {
                    n19071 = local read "Ch2_srv1_counter DI"() -> (w23429:bool)
                    n19072 = case shown="False" w23429 {
                      frame False {
                        n19073 = stacked-sequence {
                          frame #0 {
                            n19074 = while {
                              stop <- w23433 stop-if-true
                              n19075 = local read "Ch2_srv1_counter DI"() -> (w23435:bool)
                              n19076 = Wait Until Next ms Multiple(millisecond multiple=u32 100) -> ()  [unwired: 1 out]
                              n19077 = case shown="True" w23435 {
                                tunnel: [FALSE TRUE] -> w23431
                                frame False {
                                }
                                frame True {
                                }
                              }
                              n19078 = local read "position"() -> (w23434:bool)
                              n19079 = Not(x=w23434) -> (.not. x?=w23432:bool)
                              n19080 = Or(x=w23431, y=w23432) -> (x .or. y?=w23433:bool)
                            }
                          }
                          frame #1 {
                            n19081 = while {
                              stop <- w23438 stop-if-true
                              n19082 = local read "Ch2_srv1_counter DI"() -> (w23444:bool)
                              n19083 = Wait Until Next ms Multiple(millisecond multiple=u32 100) -> ()  [unwired: 1 out]
                              n19084 = case shown="False" w23444 {
                                tunnel: [TRUE FALSE] -> w23441
                                frame False {
                                n19085 = local write "CH2_Motor DO"(FALSE ("CH1_Motor DO")) -> ()
                                }
                                frame True {
                                }
                              }
                              n19086 = local read "position"() -> (w23443:bool)
                              n19087 = Not(x=w23443) -> (.not. x?=w23442:bool)
                              n19088 = Or(x=w23441, y=w23442) -> (x .or. y?=w23438:bool)
                              n19089 = Not(x=w23438) -> (.not. x?=w23439:bool)
                              n19090 = local write "CH2_Motor DO"(w23439) -> ()
                            }
                          }
                        }
                      }
                      frame True {
                        n19091 = while {
                          stop <- w23450 stop-if-true
                          n19092 = local read "Ch2_srv1_counter DI"() -> (w23448:bool)
                          n19093 = Wait Until Next ms Multiple(millisecond multiple=u32 100) -> ()  [unwired: 1 out]
                          n19094 = case shown="False" w23448 {
                            tunnel: [TRUE FALSE] -> w23452
                            frame False {
                              n19095 = local write "CH2_Motor DO"(FALSE ("CH1_Motor DO")) -> ()
                            }
                            frame True {
                            }
                          }
                          n19096 = local read "position"() -> (w23454:bool)
                          n19097 = Not(x=w23454) -> (.not. x?=w23453:bool)
                          n19098 = Or(x=w23452, y=w23453) -> (x .or. y?=w23450:bool)
                          n19099 = Not(x=w23450) -> (.not. x?=w23451:bool)
                          n19100 = local write "CH2_Motor DO"(w23451) -> ()
                        }
                      }
                    }
                  }
                  frame 3 {
                    n19101 = local read "Ch3_srv1_counter DI"() -> (w23458:bool)
                    n19102 = case shown="False" w23458 {
                      frame False {
                        n19103 = stacked-sequence {
                          frame #0 {
                            n19104 = while {
                              stop <- w23462 stop-if-true
                              n19105 = local read "Ch3_srv1_counter DI"() -> (w23464:bool)
                              n19106 = Wait Until Next ms Multiple(millisecond multiple=u32 100) -> ()  [unwired: 1 out]
                              n19107 = case shown="False" w23464 {
                                tunnel: [FALSE TRUE] -> w23460
                                frame False {
                                }
                                frame True {
                                }
                              }
                              n19108 = local read "position"() -> (w23463:bool)
                              n19109 = Not(x=w23463) -> (.not. x?=w23461:bool)
                              n19110 = Or(x=w23460, y=w23461) -> (x .or. y?=w23462:bool)
                            }
                          }
                          frame #1 {
                            n19111 = while {
                              stop <- w23467 stop-if-true
                              n19112 = local read "Ch3_srv1_counter DI"() -> (w23473:bool)
                              n19113 = Wait Until Next ms Multiple(millisecond multiple=u32 100) -> ()  [unwired: 1 out]
                              n19114 = case shown="False" w23473 {
                                tunnel: [TRUE FALSE] -> w23470
                                frame False {
                                n19115 = local write "CH3_Motor DO"(FALSE ("CH1_Motor DO")) -> ()
                                }
                                frame True {
                                }
                              }
                              n19116 = local read "position"() -> (w23472:bool)
                              n19117 = Not(x=w23472) -> (.not. x?=w23471:bool)
                              n19118 = Or(x=w23470, y=w23471) -> (x .or. y?=w23467:bool)
                              n19119 = Not(x=w23467) -> (.not. x?=w23468:bool)
                              n19120 = local write "CH3_Motor DO"(w23468) -> ()
                            }
                          }
                        }
                      }
                      frame True {
                        n19121 = while {
                          stop <- w23479 stop-if-true
                          n19122 = local read "Ch3_srv1_counter DI"() -> (w23477:bool)
                          n19123 = Wait Until Next ms Multiple(millisecond multiple=u32 100) -> ()  [unwired: 1 out]
                          n19124 = case shown="False" w23477 {
                            tunnel: [TRUE FALSE] -> w23481
                            frame False {
                              n19125 = local write "CH3_Motor DO"(FALSE ("CH1_Motor DO")) -> ()
                            }
                            frame True {
                            }
                          }
                          n19126 = local read "position"() -> (w23483:bool)
                          n19127 = Not(x=w23483) -> (.not. x?=w23482:bool)
                          n19128 = Or(x=w23481, y=w23482) -> (x .or. y?=w23479:bool)
                          n19129 = Not(x=w23479) -> (.not. x?=w23480:bool)
                          n19130 = local write "CH3_Motor DO"(w23480) -> ()
                        }
                      }
                    }
                  }
                  frame 4 {
                    n19131 = local read "Ch4_srv1_counter DI"() -> (w23487:bool)
                    n19132 = case shown="False" w23487 {
                      frame False {
                        n19133 = stacked-sequence {
                          frame #0 {
                            n19134 = while {
                              stop <- w23491 stop-if-true
                              n19135 = local read "Ch4_srv1_counter DI"() -> (w23493:bool)
                              n19136 = Wait Until Next ms Multiple(millisecond multiple=u32 100) -> ()  [unwired: 1 out]
                              n19137 = case shown="True" w23493 {
                                tunnel: [FALSE TRUE] -> w23489
                                frame False {
                                }
                                frame True {
                                }
                              }
                              n19138 = local read "position"() -> (w23492:bool)
                              n19139 = Not(x=w23492) -> (.not. x?=w23490:bool)
                              n19140 = Or(x=w23489, y=w23490) -> (x .or. y?=w23491:bool)
                            }
                          }
                          frame #1 {
                            n19141 = while {
                              stop <- w23496 stop-if-true
                              n19142 = local read "Ch4_srv1_counter DI"() -> (w23502:bool)
                              n19143 = Wait Until Next ms Multiple(millisecond multiple=u32 100) -> ()  [unwired: 1 out]
                              n19144 = case shown="False" w23502 {
                                tunnel: [TRUE FALSE] -> w23499
                                frame False {
                                n19145 = local write "CH4_Motor DO"(FALSE ("CH1_Motor DO")) -> ()
                                }
                                frame True {
                                }
                              }
                              n19146 = local read "position"() -> (w23501:bool)
                              n19147 = Not(x=w23501) -> (.not. x?=w23500:bool)
                              n19148 = Or(x=w23499, y=w23500) -> (x .or. y?=w23496:bool)
                              n19149 = Not(x=w23496) -> (.not. x?=w23497:bool)
                              n19150 = local write "CH4_Motor DO"(w23497) -> ()
                            }
                          }
                        }
                      }
                      frame True {
                        n19151 = while {
                          stop <- w23508 stop-if-true
                          n19152 = local read "Ch4_srv1_counter DI"() -> (w23506:bool)
                          n19153 = Wait Until Next ms Multiple(millisecond multiple=u32 100) -> ()  [unwired: 1 out]
                          n19154 = case shown="False" w23506 {
                            tunnel: [TRUE FALSE] -> w23510
                            frame False {
                              n19155 = local write "CH4_Motor DO"(FALSE ("CH1_Motor DO")) -> ()
                            }
                            frame True {
                            }
                          }
                          n19156 = local read "position"() -> (w23512:bool)
                          n19157 = Not(x=w23512) -> (.not. x?=w23511:bool)
                          n19158 = Or(x=w23510, y=w23511) -> (x .or. y?=w23508:bool)
                          n19159 = Not(x=w23508) -> (.not. x?=w23509:bool)
                          n19160 = local write "CH4_Motor DO"(w23509) -> ()
                        }
                      }
                    }
                  }
                }
              }
            }
          }
          frame #7 {
            n19161 = local read "position"() -> (w23516:bool)
            n19162 = case shown="True" w23516 {
              frame False {
              }
              frame True {
                n19163 = flat-sequence {
                  frame #0 {
                    w23518 = FALSE
                    n19164 = local write "Tension_Controllers_Start/Stop DO"(w23518) -> ()
                    n19165 = local write "CH1_Motor DO"(w23518) -> ()
                    n19166 = local write "CH2_Motor DO"(w23518) -> ()
                    n19167 = local write "CH3_Motor DO"(w23518) -> ()
                    n19168 = local write "CH4_Motor DO"(w23518) -> ()
                    n19169 = Wait (ms)(milliseconds to wait=u32 100) -> ()  [unwired: 1 out]
                  }
                  frame #1 {
                    n19170 = local write "Roll Forw"(TRUE ("Roll Forw")) -> ()
                  }
                  frame #2 {
                    n19171 = Wait (ms)(milliseconds to wait=u32 300) -> ()  [unwired: 1 out]
                  }
                  frame #3 {
                    n19172 = local write "TC parameter set"(TRUE ("TC parameter set")) -> ()
                  }
                  frame #4 {
                    n19173 = Wait (ms)(milliseconds to wait=u32 300) -> ()  [unwired: 1 out]
                  }
                }
              }
            }
          }
          frame #8 {
            n19174 = local read "position"() -> (w23523:bool)
            n19175 = case shown="True" w23523 {
              frame False {
              }
              frame True {
                n19176 = while {
                  i -> [w23529]
                  stop <- w23527 stop-if-true
                  n19177 = Wait Until Next ms Multiple(millisecond multiple=u32 300) -> ()  [unwired: 1 out]
                  n19178 = local read "TC parameter set"() -> (w23533:bool)
                  n19179 = local read "position"() -> (w23525:bool)
                  n19180 = local read "ABORT"() -> (w23531:bool)
                  n19181 = Not(x=w23533) -> (.not. x?=w23530:bool)
                  n19182 = Not(x=w23525) -> (.not. x?=w23524:bool)
                  n19183 = Greater Or Equal?(x=w23529, y=u32 400 ("millisecond multiple")) -> (x >= y?=w23526:bool)
                  n19184 = Compound Arithmetic op=OR(w23526, w23530, w23531, w23524) -> (w23527:bool)
                  n19185 = local write "roll error"(w23526) -> ()
                }
              }
            }
          }
          frame #9 {
            n19186 = local read "position"() -> (w23534:bool)
            n19187 = case shown="True" w23534 {
              frame False {
              }
              frame True {